vi "Configured Acquisition Trigger (Host).vi"() -> ()   [LabVIEW 2021]
doc: "Use this VI as a template to design an application that acquires data using advanced triggering logic from the NI PXIe-5170R/5171R."
uses:
  Controls/Queue_Data_Type.ctl
  <instrlib>/HSAI-RIO/Types/v1/Host/Typedefs/Temp Source.ctl
  <vilib>/FPGAPlugInAG/PXIe-5172 (8CH - 325T)/niLvFpga_Open_PXIe-5172 (8CH - 325T).vi
  <vilib>/rvi/interface/common/dynamic/niFpgaDynamicAddResources.vi
  <vilib>/FPGAPlugInAG/Dynamic/niLvFpga_Close_Dynamic.vi
  <vilib>/rvi/interface/nirviOpenFPGA/nirviOpenFPGA.xnode
  FPGA Bitfiles/Multirecord Acquisition_20220927.lvbitx
  <vilib>/rvi/interface/nirviCloseFPGA/nirviCloseFPGA.xnode
  Device Session/Device Session.lvclass
  <instrlib>/HSAI-RIO/Types/v1/Host/niHSAI Types v1 Host.lvlib
  <vilib>/Utility/TDMS File Viewer/NI_TDMS File Viewer.lvlib
panel:
  out "error out 2":errorcluster
  out "appended path":path
  out "Trigger":bool
  in  "trigger level lo (V)":dbl=-0.25
  in  "trigger level hi (V)":dbl=0.25
  out "actual sample rate":dbl=200000000.0 format="%#_6p"
  in  "onboard sample clock rate":dbl(ring)=200000000.0 items=["250 MHz"=250000000.0, "200 MHz"=200000000.0, "150 MHz"=150000000.0]
  in  "impedance":enum8{"Default", "1 mega ohm", "50 ohm"}(ring)=enum."50 ohm"
  in  "vertical offset (V)":dbl format="%.2p"
  out "Graph":T1(graph)=[{"relativeX"=-2.5e-06, "sample rate"=5e-09, "data in"=[0.6086595323350694, 0.6082560221354166, 0.606594509548611, 0.6064046223958333, 0.6059061686197916, 0.6071879069010416, 0.6087544759114583, 0.6111043294270833, 0.6109144422743055, 0.6111043294270833, 0.6073777940538194, 0.6095377604166666, 0.6135491265190971, 0.606594509548611, 0.6074727376302083, 0.610012478298611, 0.6123860677083333, 0.6079711914062499, 0.613857693142361, 0.6101311577690971, 0.6120775010850694, 0.6082560221354166, 0.6126708984374999, 0.6097276475694444, 0.6118876139322916, 0.6109144422743055, 0.6097276475694444, 0.6128607855902777, 0.6109144422743055, 0.6095377604166666, 0.6115790473090277, 0.6128607855902777, 0.6139526367187499, 0.6110093858506944, 0.609157986111111, 0.6076863606770833, 0.6129557291666666, 0.6110093858506944, 0.6092529296874999, 0.6120775010850694, 0.6131693522135416, 0.6108194986979166, 0.6126708984374999, 0.6101311577690971, 0.6068793402777777, 0.6114841037326388, 0.6140475802951388, 0.6120775010850694, 0.6108194986979166, 0.6083509657118055, 0.610226101345486, 0.6116977267795138, 0.6115790473090277, 0.6137627495659721, 0.611294216579861, 0.6116977267795138, 0.6105109320746527, 0.6104159884982638, 0.6079711914062499, 0.6094428168402777, 0.6128607855902777, 0.6097276475694444, 0.6101311577690971, 0.6093478732638888, 0.6140475802951388, 0.612575954861111, 0.6087544759114583, 0.6094428168402777, 0.6104159884982638, 0.6115790473090277, 0.6072828504774305, 0.6098225911458333, 0.608944363064236, 0.6110093858506944, 0.6075676812065971, 0.607876247829861, 0.6092529296874999, 0.6094428168402777, 0.610226101345486, 0.6118876139322916, 0.6116977267795138, 0.6086595323350694, 0.6096327039930555, 0.6072828504774305, 0.6073777940538194, 0.6075676812065971, 0.6118876139322916, 0.6074727376302083, 0.6069742838541666, 0.6045294867621527, 0.6111043294270833, 0.6067843967013888, 0.611294216579861, 0.6122911241319444, 0.6107245551215277, 0.6080661349826388, 0.6068793402777777, 0.6088494194878471, 0.6104159884982638, 0.6105109320746527, 0.6124810112847221, 0.6080661349826388, 0.6104159884982638, 0.611294216579861, 0.6111992730034721, 0.6072828504774305, 0.6110093858506944, 0.6111043294270833, 0.6119825575086805, 0.6111043294270833, 0.6110093858506944, 0.6121961805555555, 0.612575954861111, 0.6108194986979166, 0.6104159884982638, 0.6071879069010416, 0.6103210449218749, 0.6103210449218749, 0.6147359212239583, 0.6121961805555555, 0.6114841037326388, 0.6064046223958333, 0.6093478732638888, 0.6081610785590277, 0.610012478298611, 0.6083509657118055, 0.610226101345486, 0.6092529296874999, 0.6120775010850694, 0.6103210449218749, 0.6119825575086805, 0.6126708984374999, 0.6122911241319444, 0.6142374674479166, 0.6115790473090277, 0.6158989800347221, 0.6111043294270833, 0.607876247829861, 0.6103210449218749, 0.608944363064236, 0.6142374674479166, 0.6111043294270833, 0.6123860677083333, 0.609157986111111, 0.6096327039930555, 0.6071879069010416, 0.6084459092881944, 0.6116977267795138, 0.610226101345486, 0.6099175347222221, 0.6082560221354166, 0.6098225911458333, 0.6087544759114583, 0.6098225911458333, 0.6107245551215277, 0.6093478732638888, 0.6111043294270833, 0.6122911241319444, 0.610226101345486, 0.6118876139322916, 0.6081610785590277, 0.6081610785590277, 0.6082560221354166, 0.6040547688802083, 0.6075676812065971, 0.6070929633246527, 0.6083509657118055, 0.6111992730034721, 0.6106058756510416, 0.6114841037326388, 0.6104159884982638, 0.6143324110243055, 0.6117926703559027, 0.6116977267795138, 0.6123860677083333, 0.6122911241319444, 0.6105109320746527, 0.6088494194878471, 0.6123860677083333, 0.6086595323350694, 0.6127658420138888, 0.6090393066406249, 0.6109144422743055, 0.6122911241319444, 0.6094428168402777, 0.6077813042534721, 0.6071879069010416, 0.609157986111111, 0.6092529296874999, 0.6090393066406249, 0.6086595323350694, 0.6050279405381944, 0.6086595323350694, 0.6076863606770833, 0.6061197916666666, 0.606594509548611, 0.6097276475694444, 0.6101311577690971, 0.6088494194878471, 0.610012478298611, 0.6081610785590277, 0.6057162814670138, 0.6113891601562499, 0.6087544759114583, 0.6080661349826388, 0.6113891601562499, 0.6132642957899305, 0.6108194986979166, 0.6114841037326388, 0.609157986111111, 0.6077813042534721, 0.6077813042534721, 0.6146172417534721, 0.6084459092881944, 0.6111992730034721, 0.6080661349826388, 0.6088494194878471, 0.6054077148437499, 0.6085408528645833, 0.6049329969618055, 0.6075676812065971, 0.6104159884982638, 0.6104159884982638, 0.6111992730034721, 0.6096327039930555, 0.6064995659722221, 0.6051228841145833, 0.6067843967013888, 0.602962917751736, 0.6096327039930555, 0.6083509657118055, 0.6070929633246527, 0.6074727376302083, 0.6121961805555555, 0.6122911241319444, 0.6092529296874999, 0.6139526367187499, 0.6120775010850694, 0.6110093858506944, 0.6107245551215277, 0.6132642957899305, 0.607876247829861, 0.607876247829861, 0.6051228841145833, 0.6093478732638888, 0.6070929633246527, 0.6110093858506944, 0.609157986111111, 0.6084459092881944, 0.6097276475694444, 0.6155192057291666, 0.6103210449218749, 0.6086595323350694, 0.6117926703559027, 0.6099175347222221, 0.6132642957899305, 0.6084459092881944, 0.6081610785590277, 0.6067843967013888, 0.6096327039930555, 0.6114841037326388, 0.6119825575086805, 0.6075676812065971, 0.6109144422743055, 0.6129557291666666, 0.610226101345486, 0.6121961805555555, 0.6137627495659721, 0.6111043294270833, 0.609157986111111, 0.6092529296874999, 0.6109144422743055, 0.6064046223958333, 0.6070929633246527, 0.6093478732638888, 0.6097276475694444, 0.6115790473090277, 0.6118876139322916, 0.6106058756510416, 0.6135491265190971, 0.6126708984374999, 0.6079711914062499, 0.6103210449218749, 0.6101311577690971, 0.6105109320746527, 0.6120775010850694, 0.6088494194878471, 0.6097276475694444, 0.6120775010850694, 0.6080661349826388, 0.6108194986979166, 0.6123860677083333, 0.6104159884982638, 0.6120775010850694, 0.6126708984374999, 0.6094428168402777, 0.6120775010850694, 0.6115790473090277, 0.6123860677083333, 0.6104159884982638, 0.6093478732638888, 0.6097276475694444, 0.6098225911458333, 0.6056213378906249, 0.6108194986979166, 0.607876247829861, 0.6111992730034721, 0.6082560221354166, 0.6082560221354166, 0.6106058756510416, 0.608944363064236, 0.6094428168402777, 0.6071879069010416, 0.608944363064236, 0.6062147352430555, 0.6075676812065971, 0.6097276475694444, 0.6114841037326388, 0.6072828504774305, 0.608944363064236, 0.6093478732638888, 0.6084459092881944, 0.6101311577690971, 0.6056213378906249, 0.611294216579861, 0.6083509657118055, 0.6097276475694444, 0.6085408528645833, 0.6116977267795138, 0.6109144422743055, 0.6111043294270833, 0.6098225911458333, 0.613857693142361, 0.6115790473090277, 0.6121961805555555, 0.6096327039930555, 0.6124810112847221, 0.6115790473090277, 0.6116977267795138, 0.610226101345486, 0.6124810112847221, 0.6154242621527777, 0.6110093858506944, 0.6092529296874999, 0.6106058756510416, 0.608944363064236, 0.6104159884982638, 0.6085408528645833, 0.6140475802951388, 0.6097276475694444, 0.609157986111111, 0.6077813042534721, 0.6055026584201388, 0.6095377604166666, 0.6147359212239583, 0.6115790473090277, 0.6111043294270833, 0.6101311577690971, 0.6090393066406249, 0.6103210449218749, 0.611294216579861, 0.6083509657118055, 0.6143324110243055, 0.6121961805555555, 0.6111043294270833, 0.608944363064236, 0.6116977267795138, 0.6120775010850694, 0.610226101345486, 0.6145222981770833, 0.612575954861111, 0.6137627495659721, 0.6104159884982638, 0.6120775010850694, 0.6107245551215277, 0.610226101345486, 0.6134541829427083, 0.6116977267795138, 0.6153293185763888, 0.6103210449218749, 0.6118876139322916, 0.6080661349826388, 0.6124810112847221, 0.6108194986979166, 0.6118876139322916, 0.6106058756510416, 0.6106058756510416, 0.6144273546006944, 0.6127658420138888, 0.612575954861111, 0.608944363064236, 0.6111043294270833, 0.6099175347222221, 0.613644070095486, 0.6150207519531249, 0.6147359212239583, 0.613857693142361, 0.6097276475694444, 0.6118876139322916, 0.6046481662326388, 0.6111043294270833, 0.6098225911458333, 0.608944363064236, 0.607876247829861, 0.611294216579861, 0.6132642957899305, 0.611294216579861, 0.6088494194878471, 0.610226101345486, 0.6087544759114583, 0.6129557291666666, 0.6056213378906249, 0.6119825575086805, 0.6096327039930555, 0.6135491265190971, 0.6062147352430555, 0.608944363064236, 0.6101311577690971, 0.6132642957899305, 0.6090393066406249, 0.6128607855902777, 0.6093478732638888, 0.6105109320746527, 0.6064046223958333, 0.6095377604166666, 0.6085408528645833, 0.610226101345486, 0.6101311577690971, 0.6101311577690971, 0.6126708984374999, 0.6096327039930555, 0.6105109320746527, 0.6121961805555555, 0.6116977267795138, 0.6118876139322916, 0.6096327039930555, 0.6105109320746527, 0.6106058756510416, 0.6096327039930555, 0.6092529296874999, 0.6110093858506944, 0.612575954861111, 0.613644070095486, 0.6094428168402777, 0.6117926703559027, 0.610012478298611, 0.612575954861111, 0.6107245551215277, 0.6111992730034721, 0.6109144422743055, 0.6067843967013888, 0.6051228841145833, 0.6072828504774305, 0.6062147352430555, 0.6080661349826388, 0.6107245551215277, 0.6160888671874999, 0.6103210449218749, 0.6114841037326388, 0.6113891601562499, 0.6104159884982638, 0.609157986111111, 0.6092529296874999, 0.6064995659722221, 0.6106058756510416, 0.6117926703559027, 0.6117926703559027, 0.6141425238715277, 0.6099175347222221, 0.6096327039930555, 0.6127658420138888, 0.6131693522135416, 0.6105109320746527, 0.6119825575086805, 0.6128607855902777, 0.6081610785590277, 0.6085408528645833, 0.6099175347222221, 0.611294216579861, 0.610012478298611, 0.6103210449218749, 0.6071879069010416, 0.611294216579861, 0.6051228841145833, 0.6084459092881944, 0.6082560221354166, 0.6124810112847221, 0.6109144422743055, 0.6108194986979166, 0.6131693522135416, 0.6107245551215277, 0.6119825575086805, 0.6121961805555555, 0.6143324110243055, 0.6114841037326388, 0.6115790473090277, 0.6164923773871527, 0.6106058756510416, 0.6109144422743055, 0.6116977267795138, 0.6084459092881944, 0.6106058756510416, 0.6081610785590277, 0.605312771267361, 0.6081610785590277, 0.6066894531249999, 0.608944363064236, 0.607876247829861, 0.6111043294270833, 0.6109144422743055, 0.6116977267795138, 0.6137627495659721, 0.6117926703559027, 0.6099175347222221, 0.6083509657118055, 0.6094428168402777, 0.6105109320746527, 0.6085408528645833, 0.6107245551215277, 0.610226101345486, 0.6118876139322916, 0.608944363064236, 0.6123860677083333, 0.6099175347222221, 0.610226101345486, 0.6055026584201388, 0.612575954861111, 0.6115790473090277, 0.6109144422743055, 0.6079711914062499, 0.6111043294270833, 0.6072828504774305, 0.610012478298611, 0.6083509657118055, 0.611294216579861, 0.6070929633246527, 0.6119825575086805, 0.6094428168402777, 0.6123860677083333, 0.6115790473090277, 0.6113891601562499, 0.6122911241319444, 0.6099175347222221, 0.6111992730034721, 0.6108194986979166, 0.6110093858506944, 0.6084459092881944, 0.6066894531249999, 0.6057162814670138, 0.6084459092881944, 0.6116977267795138, 0.6090393066406249, 0.610226101345486, 0.6104159884982638, 0.6087544759114583, 0.6094428168402777, 0.6088494194878471, 0.6081610785590277, 0.6119825575086805, 0.6101311577690971, 0.610226101345486, 0.6079711914062499, 0.6119825575086805, 0.6092529296874999, 0.6113891601562499, 0.609157986111111, 0.6064046223958333, 0.6076863606770833, 0.6114841037326388, 0.609157986111111, 0.6116977267795138, 0.6082560221354166, 0.6097276475694444, 0.6093478732638888, 0.6132642957899305, 0.6124810112847221, 0.6123860677083333, 0.6115790473090277, 0.6152343749999999, 0.610226101345486, 0.6103210449218749, 0.6081610785590277, 0.6095377604166666, 0.6054077148437499, 0.6068793402777777, 0.606594509548611, 0.612575954861111, 0.6058112250434027, 0.6124810112847221, 0.6048380533854166, 0.612575954861111, 0.6095377604166666, 0.6135491265190971, 0.6095377604166666, 0.612575954861111, 0.6106058756510416, 0.6117926703559027, 0.6121961805555555, 0.6117926703559027, 0.6086595323350694, 0.6104159884982638, 0.610012478298611, 0.609157986111111, 0.6093478732638888, 0.6111043294270833, 0.6081610785590277, 0.6088494194878471, 0.6088494194878471, 0.6077813042534721, 0.6070929633246527, 0.605312771267361, 0.6068793402777777, 0.6118876139322916, 0.6097276475694444, 0.6116977267795138, 0.6073777940538194, 0.610012478298611, 0.6072828504774305, 0.6090393066406249, 0.6052178276909721, 0.6084459092881944, 0.604244656032986, 0.6098225911458333, 0.6103210449218749, 0.610012478298611, 0.6104159884982638, 0.6134541829427083, 0.6114841037326388, 0.6140475802951388, 0.6126708984374999, 0.607876247829861, 0.6103210449218749, 0.6132642957899305, 0.6106058756510416, 0.6113891601562499, 0.6064995659722221, 0.6111043294270833, 0.6099175347222221, 0.6099175347222221, 0.6094428168402777, 0.6144273546006944, 0.6113891601562499, 0.611294216579861, 0.6124810112847221, 0.6123860677083333, 0.6152343749999999, 0.6124810112847221, 0.6121961805555555, 0.6115790473090277, 0.6141425238715277, 0.6096327039930555, 0.6107245551215277, 0.6081610785590277, 0.6098225911458333, 0.6099175347222221, 0.6057162814670138, 0.6074727376302083, 0.6086595323350694, 0.6123860677083333, 0.6122911241319444, 0.6122911241319444, 0.6103210449218749, 0.6101311577690971, 0.6050279405381944, 0.6057162814670138, 0.608944363064236, 0.6116977267795138, 0.6064995659722221, 0.6126708984374999, 0.606594509548611, 0.608944363064236, 0.606594509548611, 0.6114841037326388, 0.6087544759114583, 0.6093478732638888, 0.6087544759114583, 0.6095377604166666, 0.6064995659722221, 0.6120775010850694, 0.6103210449218749, 0.6147359212239583, 0.6122911241319444, 0.6110093858506944, 0.6088494194878471, 0.6081610785590277, 0.6074727376302083, 0.608944363064236, 0.6055026584201388, 0.6145222981770833, 0.6116977267795138, 0.6123860677083333, 0.610226101345486, 0.6114841037326388, 0.6121961805555555, 0.6135491265190971, 0.6095377604166666, 0.6082560221354166, 0.6067843967013888, 0.610012478298611, 0.6075676812065971, 0.6133592393663194, 0.610012478298611, 0.6145222981770833, 0.6126708984374999, 0.6143324110243055, 0.6122911241319444, 0.6093478732638888, 0.6062147352430555, 0.6059061686197916, 0.6033664279513888, 0.6051228841145833, 0.6071879069010416, 0.6094428168402777, 0.611294216579861, 0.6101311577690971, 0.6095377604166666, 0.6087544759114583, 0.6115790473090277, 0.6147359212239583, 0.6104159884982638, 0.6131693522135416, 0.610012478298611, 0.6081610785590277, 0.6067843967013888, 0.6087544759114583, 0.6061197916666666, 0.6084459092881944, 0.6104159884982638, 0.6119825575086805, 0.6111992730034721, 0.6105109320746527, 0.6086595323350694, 0.6086595323350694, 0.6098225911458333, 0.6111992730034721, 0.6076863606770833, 0.6132642957899305, 0.6084459092881944, 0.6096327039930555, 0.6086595323350694, 0.6124810112847221, 0.607876247829861, 0.6088494194878471, 0.6092529296874999, 0.6123860677083333, 0.6109144422743055, 0.6114841037326388, 0.6126708984374999, 0.6106058756510416, 0.6092529296874999, 0.6084459092881944, 0.6072828504774305, 0.6086595323350694, 0.6062147352430555, 0.6115790473090277, 0.6127658420138888, 0.6150207519531249, 0.6126708984374999, 0.614925808376736, 0.6139526367187499, 0.615993923611111, 0.6079711914062499, 0.6122911241319444, 0.6107245551215277, 0.6153293185763888, 0.6120775010850694, 0.611294216579861, 0.6111992730034721, 0.6130506727430555, 0.6116977267795138, 0.6097276475694444, 0.6066894531249999, 0.6093478732638888, 0.6087544759114583, 0.610012478298611, 0.6098225911458333, 0.6131693522135416, 0.6123860677083333, 0.6124810112847221, 0.6087544759114583, 0.6095377604166666, 0.6077813042534721, 0.6076863606770833, 0.6060011121961805, 0.610012478298611, 0.610012478298611, 0.6103210449218749, 0.6142374674479166, 0.6153293185763888, 0.616207546657986, 0.6110093858506944, 0.6132642957899305, 0.6129557291666666, 0.611294216579861, 0.6103210449218749, 0.6098225911458333, 0.6113891601562499, 0.6094428168402777, 0.6098225911458333, 0.6111992730034721, 0.6128607855902777, 0.6128607855902777, 0.611294216579861, 0.6123860677083333, 0.6127658420138888, 0.6094428168402777, 0.6068793402777777, 0.6068793402777777, 0.6107245551215277, 0.6083509657118055, 0.613644070095486, 0.607876247829861, 0.6115790473090277, 0.6097276475694444, 0.6109144422743055, 0.6101311577690971, 0.6115790473090277, 0.6145222981770833, 0.6116977267795138, 0.6062147352430555, 0.6086595323350694, 0.6107245551215277, 0.6098225911458333, 0.6145222981770833, 0.6119825575086805, 0.6148308648003471, 0.6113891601562499, 0.6070929633246527, 0.6067843967013888, 0.6062147352430555, 0.6090393066406249, 0.6079711914062499, 0.6090393066406249, 0.6101311577690971, 0.6130506727430555, 0.6116977267795138, 0.6103210449218749, 0.6079711914062499, 0.6067843967013888, 0.6086595323350694, 0.6090393066406249, 0.6087544759114583, 0.6090393066406249, 0.6104159884982638, 0.6083509657118055, 0.6124810112847221, 0.6110093858506944, 0.6107245551215277, 0.6120775010850694, 0.6090393066406249, 0.6090393066406249, 0.6099175347222221, 0.6103210449218749, 0.6073777940538194, 0.611294216579861, 0.6086595323350694, 0.6103210449218749, 0.6121961805555555, 0.6109144422743055, 0.6087544759114583, 0.610012478298611, 0.6045294867621527, 0.6064995659722221, 0.6036512586805555, 0.6101311577690971, 0.6092529296874999, 0.6107245551215277, 0.6092529296874999, 0.6148308648003471, 0.6101311577690971, 0.6092529296874999, 0.6062147352430555, 0.6069742838541666, 0.6090393066406249, 0.6070929633246527, 0.6111043294270833, 0.6101311577690971, 0.6114841037326388, 0.6147359212239583, 0.6148308648003471, 0.6143324110243055, 0.6135491265190971, 0.6122911241319444, 0.6106058756510416, 0.6115790473090277, 0.6114841037326388, 0.6130506727430555, 0.6094428168402777, 0.608944363064236, 0.6101311577690971, 0.6077813042534721, 0.6093478732638888, 0.6122911241319444, 0.6094428168402777, 0.6145222981770833, 0.6093478732638888, 0.610012478298611, 0.6114841037326388, 0.6109144422743055, 0.6104159884982638, 0.610226101345486, 0.6097276475694444, 0.6093478732638888, 0.6117926703559027, 0.6146172417534721, 0.610012478298611, 0.611294216579861, 0.6110093858506944, 0.6127658420138888, 0.6131693522135416, 0.6104159884982638, 0.6129557291666666, 0.6095377604166666, 0.6069742838541666, 0.6118876139322916, 0.6093478732638888, 0.6099175347222221, 0.6120775010850694, 0.6119825575086805, 0.6139526367187499, 0.6084459092881944, 0.6092529296874999, 0.6116977267795138, 0.6070929633246527, 0.6086595323350694, 0.610012478298611, 0.6087544759114583, 0.6064046223958333, 0.6108194986979166, 0.6069742838541666, 0.6139526367187499, 0.6088494194878471, 0.6108194986979166, 0.6143324110243055, 0.613644070095486, 0.6088494194878471, 0.6123860677083333, 0.6110093858506944, 0.6153293185763888, 0.6076863606770833, 0.6103210449218749, 0.607876247829861, 0.6119825575086805, 0.6077813042534721, 0.6116977267795138, 0.6106058756510416, 0.6137627495659721, 0.6113891601562499, 0.6093478732638888, 0.6062147352430555, 0.6093478732638888, 0.6123860677083333, 0.6104159884982638, 0.6124810112847221, 0.6155192057291666, 0.613857693142361, 0.6114841037326388, 0.6098225911458333, 0.6127658420138888, 0.6086595323350694, 0.6085408528645833, 0.6054077148437499, 0.6104159884982638, 0.6064995659722221, 0.611294216579861, 0.6092529296874999, 0.612575954861111, 0.6134541829427083, 0.6097276475694444, 0.6099175347222221, 0.6108194986979166, 0.6097276475694444, 0.614925808376736, 0.6132642957899305, 0.6154242621527777, 0.6142374674479166, 0.6120775010850694, 0.6118876139322916, 0.6128607855902777, 0.611294216579861, 0.6103210449218749, 0.6072828504774305, 0.6105109320746527, 0.6058112250434027, 0.607876247829861, 0.6148308648003471, 0.6115790473090277, 0.6101311577690971, 0.6106058756510416, 0.6074727376302083, 0.6107245551215277, 0.6127658420138888, 0.6098225911458333, 0.6095377604166666, 0.6088494194878471, 0.6113891601562499, 0.6153293185763888, 0.6110093858506944, 0.6119825575086805, 0.6080661349826388]}, ...(2 in all)]
  out "fpga temperature (°C)":dbl(slide)=84.16040039062506 scale=0.0..96.0 scale format="%#_6p"
  out "power consumption (W)":dbl(slide)=28.75 scale=0.0..38.25 scale format="%#_6p"
  in  "decimation factor":u16=1
  in  "coupling":enum8{"Default", "DC", "AC"}(ring)
  in  "bandwidth":T2(ring)
  in  "pretrigger samples":u64=500
  in  "number of samples":u64=1000
  in  "RIO Device":tag="PXI1Slot2"
  in  "channel(s)":string="0,1"
  in  "vertical range (Vpp)":dbl=1.0 format="%.2p"
  out "error out":errorcluster
  in  "stop":bool
  # "RIO Device"
  # "Vertical Settings"
  # "Trigger Settings"
  # "System Monitor"
  # "Acquisition Settings"
  # "Clocking"
  # "DSP"
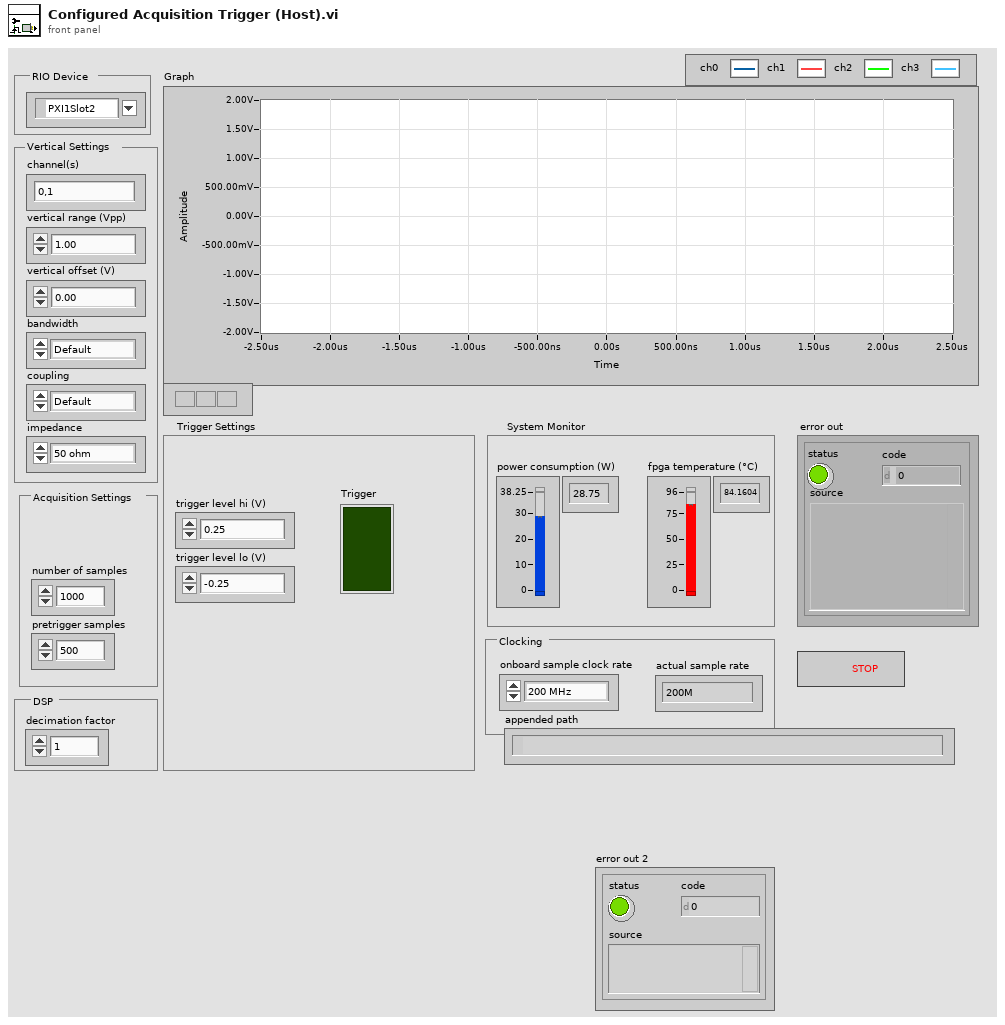
[diagram p1: front panel]
types:
  T1 = cluster{"relativeX":dbl, "sample rate":dbl, "data in":dbl[]}[]
  T2 = enum8{"Default", "Full Bandwidth", "Anti-alias Filter", "80 MHz FIR Filter", "40 MHz FIR Filter", "20 MHz FIR Filter"}
  T3 = enum16{"Immediate", "A", "B", "OR", "AND", "A THEN B", "B THEN A", "High Resolution"}
  T4 = typedef "niHSAI Types v1 Host.lvlib/Temp Source.ctl" = enum8{"Device Temperature", "Thermal Shutdown Margin", "FPGA Temperature", "FPGA Temperature Limit"}
  T5 = typedef "Queue_Data_Type.ctl" = cluster{"date/time string":string, "data":dbl[][]}
  T6 = enum16{"open", "open or create", "create or replace", "create", "open (read-only)"}
  T7 = cluster{"date/time string":string, "data":dbl[][]}
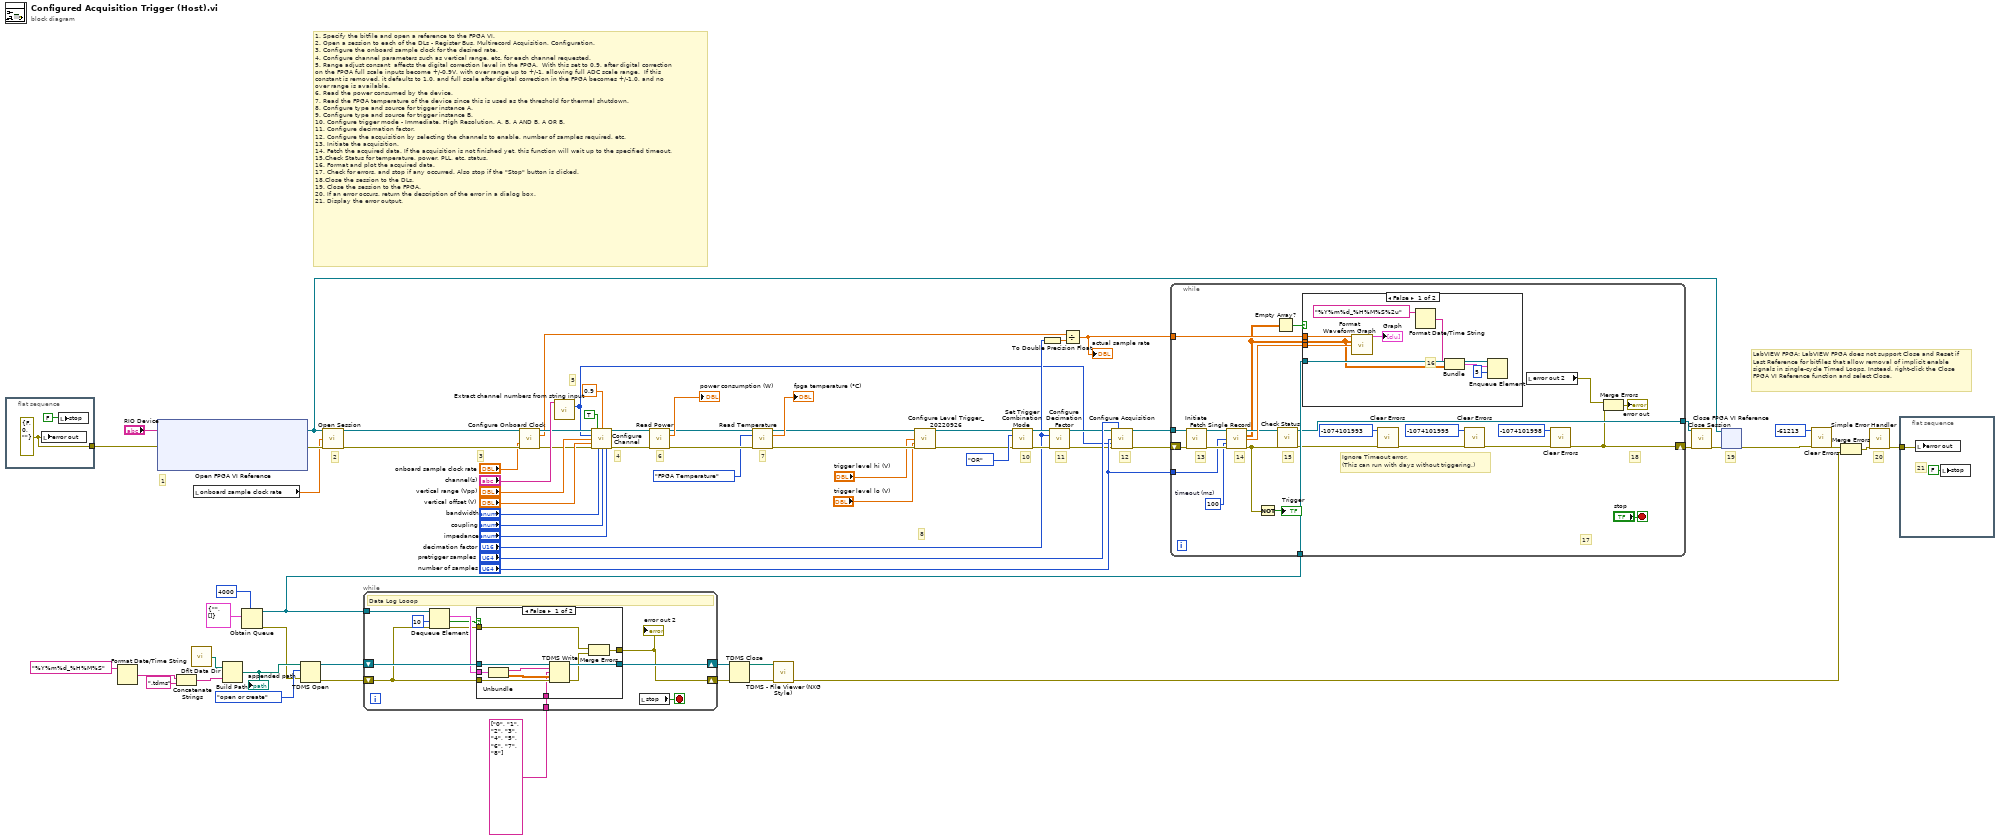
[diagram p0: block diagram]
diagram:
  # "4"
  # "5"
  # "7"
  # "6"
  # "11"
  # "3"
  # "10"
  # "8"
  # "12"
  # "LabVIEW FPGA: LabVIEW FPGA does not support Close and Reset if Last Reference for bitfiles that allow removal of implicit enable signals in single-cycle Timed Loops. Instead, right-click the Close FPGA VI Reference function and select Close."
  # "20"
  # "19"
  # "1. Specify the bitfile and open a reference to the FPGA VI.\n2. Open a session to each of the DLs - Register Bus, Multirecord Acquisition, Configuration.\n3. Configure the onboard sample clock for the desired rate.\n4. Configure channel parameters such as vertical range, etc. for each channel requested.\n5. Range adjust consant  affects the digital correction level in the FPGA.  With this set to 0.9, after digital correction\non the FPGA full scale inputs become +/-0.9V, with over range up to +/-1, allowing full ADC scale range.  If this \nconstant is removed, it defaults to 1.0, and full scale after digital correction in the FPGA becomes +/-1.0, and no\nover range is available.  \n6. Read the power consumed by the device.\n7. Read the FPGA temperature of the device since this is used as the threshold for thermal shutdown.\n8. Configure type and source for trigger instance A.\n9. Configure type and source for trigger instance B.\n10. Configure trigger mode - Immediate, High Resolution, A, B, A AND B, A OR B.\n11. Configure decimation factor.\n12. Configure the acquisition by selecting the channels to enable, number of samples required, etc.\n13. Initiate the acquisition.\n14. Fetch the acquired data. If the acquisition is not finished yet, this function will wait up to the specified timeout.\n15.Check Status for temperature, power, PLL, etc. status. \n16. Format and plot the acquired data.\n17. Check for errors, and stop if any occurred. Also stop if the \"Stop\" button is clicked.\n18.Close the session to the DLs.\n19. Close the session to the FPGA.\n20. If an error occurs, return the description of the error in a dialog box.\n21. Display the error output."
  # "2"
  # "1"
  n1 = flat-sequence {
    tunnel: [w74] -> w65
    frame #0 {
      w74 = errorcluster {"status"=FALSE, "code"=0, "source"=""} ("error out")
      n2 = local write "error out"(w74) -> ()
      n3 = local write "stop"(FALSE ("stop")) -> ()
    }
  }
  n4 = Format Date/Time String(time format string (%c)="%Y%m%d_%H%M%S") -> (date/time string=w63:string)  [unwired: 2 in]
  n5 = xnode "Open FPGA VI Reference"("error in"=w65, "resource name"="RIO Device") -> ("FPGA VI Reference Out"=w68:refnum<k20>, "error out"=w69:errorcluster)
  n6 = Concatenate Strings(w63, ".tdms" ("string")) -> (w62:string)
  n7 = call <vilib>:"Dflt Data Dir.vi"() -> ("App:Default Data Directory"=w64:path)
  n8 = local read "onboard sample clock rate"() -> (w67:dbl)
  n9 = Build Path(base path=w64, name or relative path=w62) -> (appended path=w59:path)
  "appended path" <- w59
  n10 = Obtain Queue(max queue size (-1, unlimited)=4000, element data type=T5 {"date/time string"="", "data"=[]} ("cluster")) -> (queue out=w49:refnum<queue>, error out=w57:errorcluster)  [unwired: 3 in, 1 out]
  n11 = TDMS Open(8:w57, 10:T6."open or create" ("operation (0:open)"), 11:w59) -> (0:w55:errorcluster, 3:w52:refnum<k34>)  [unwired: 4 in]
  n12 = call "Open Session.vi"("fpga reference in"=w68, "adc clock rate (Hz)"=w67, "error in"=w69) -> ("device session out"=w72:refnum<class "Device Session.lvclass">, "error out"=w71:errorcluster)  [unwired: 11 in]
  n13 = while {
    shift-right: [w77] -> w54
    shift-left: w55 -> [w82]
    shift-right: [w84] -> w51
    shift-left: w52 -> [w85]
    tunnel: w49 -> [w83]
    tunnel: string[] ["0", "1", "2", "3", "4", "5", "6", "7", "8"] ("channel name(s) in (Untitled)") -> [w75]
    stop <- w79 stop-if-true
    # "Data Log Looop"
    n14 = Dequeue Element(queue=w83, timeout in ms (-1)=10, error in (no error)=w82) -> (element=w81:T5, timed out?=w76:bool, error out=w80:errorcluster)  [unwired: 1 out]
    n15 = case shown="False" w76 {
      tunnel: w85 -> [w95 w97]
      tunnel: [w94 w97] -> w84
      tunnel: w82 -> [w93 _]
      tunnel: w81 -> [w92 _]
      tunnel: w80 -> [w91 w96]
      tunnel: [w89 w96] -> w77
      tunnel: w75 -> [w86 _]
      frame False {
        n16 = Unbundle(w92) -> ("date/time string"=w88:string, "data"=w87:dbl[][])
        n17 = TDMS Write(0:w95, 5:w88, 7:w86, 9:w87, 11:w93) -> (4:w94:refnum<k34>, 15:w90:errorcluster)  [unwired: 1 in, 2 out]
        n18 = Merge Errors(w91, w90) -> (w89:errorcluster)
      }
      frame True {
        # "Timed out. No data."
      }
    }
    "error out 2" <- w77
    n19 = local read "stop"() -> (w79:bool)
  }
  n20 = call "Configure Onboard Clock.vi"("device session in"=w72, "adc clock rate (Hz)"="onboard sample clock rate", "error in"=w71) -> ("device session out"=w34:refnum<class "Device Session.lvclass">, "actual adc clock rate (Hz)"=w26:dbl, "error out"=w33:errorcluster)  [unwired: 9 in, 1 out]
  n21 = call "Extract channel numbers from string input.vi"("channel input"="channel(s)") -> ("array of chans"=w8:u32[])  [unwired: 13 in, 1 out]
  n22 = call "Configure Channel.vi"("device session in"=w34, "enable channel (T)"=TRUE ("enable channel"), "range adjust"=0.9, "channels"=w8, "vertical range (Vpp)"="vertical range (Vpp)", "vertical offset (V)"="vertical offset (V)", "error in"=w33, "bandwidth"="bandwidth", "coupling"="coupling", "impedance"="impedance") -> ("device session out"=w20:refnum<class "Device Session.lvclass">, "error out"=w19:errorcluster)  [unwired: 4 in]
  n23 = call "Read Power.vi"("device session in"=w20, "error in"=w19) -> ("device session out"=w21:refnum<class "Device Session.lvclass">, "power (W)"=→"power consumption (W)":dbl, "error out"=w22:errorcluster)  [unwired: 11 in]
  n24 = TDMS Close(8:w54, 11:w51) -> (0:w53:errorcluster, 3:w50:path)
  n25 = call "Read Temperature.vi"("device session in"=w21, "source"=Temp_Source."FPGA Temperature", "error in"=w22) -> ("device session out"=w18:refnum<class "Device Session.lvclass">, "temperature (°C)"=→"fpga temperature (°C)":dbl, "error out"=w17:errorcluster)  [unwired: 10 in]
  n26 = call <vilib>:"TDMS - File Viewer (NXG Style).vi"("error in"=w53, "file in"=w50) -> ("error out"=w47:errorcluster)  [unwired: 8 in, 1 out]
  n27 = call "Configure Level Trigger_20220926.vi"("device session in"=w18, "trigger level hi (V)"="trigger level hi (V)", "trigger level lo (V)"="trigger level lo (V)", "error in"=w17) -> ("device session out"=w7:refnum<class "Device Session.lvclass">, "error out"=w6:errorcluster)  [unwired: 10 in]
  n28 = call "Set Trigger Combination Mode.vi"("device session in"=w7, "mode"=T3."OR", "error in"=w6) -> ("device session out"=w31:refnum<class "Device Session.lvclass">, "error out"=w30:errorcluster)  [unwired: 11 in]
  n29 = To Double Precision Float(number="decimation factor") -> (double precision float=w32:dbl)
  n30 = call "Configure Decimation Factor.vi"("device session in"=w31, "decimation factor"="decimation factor", "error in"=w30) -> ("device session out"=w28:refnum<class "Device Session.lvclass">, "error out"=w29:errorcluster)  [unwired: 11 in]
  n31 = Divide(x=w26, y=w32) -> (x/y=w10:dbl)
  "actual sample rate" <- w10
  n32 = call "Configure Acquisition.vi"("device session in"=w28, "pretrigger samples"="pretrigger samples", "number of samples"="number of samples", "channels to store"=w8, "error in"=w29) -> ("device session out"=w39:refnum<class "Device Session.lvclass">, "error out"=w40:errorcluster)  [unwired: 8 in, 1 out]
  n33 = while {
    tunnel: w49 -> [w122]
    tunnel: w39 -> [w118]
    tunnel: "number of samples" -> [w116]
    tunnel: w10 -> [w112]
    shift-right: [w98] -> w1
    shift-left: w40 -> [w121]
    tunnel: [w99] -> w3
    stop <- "stop" stop-if-true
    w117 = 100  # timeout (ms)
    # "Ignore Timeout error.\n(This can run with days without triggering.)"
    # "15"
    # "17"
    # "14"
    # "13"
    # "18"
    n34 = call "Initiate.vi"("device session in"=w118, "error in"=w121) -> ("device session out"=w119:refnum<class "Device Session.lvclass">, "error out"=w120:errorcluster)  [unwired: 12 in]
    n35 = call "Fetch Single Record.vi"("device session in"=w119, "number of samples"=w116, "timeout (ms)"=w117, "error in"=w120) -> ("device session out"=w113:refnum<class "Device Session.lvclass">, "data"=w104:dbl[][], "relativeX (samples)"=w115:dbl, "error out"=w105:errorcluster)  [unwired: 7 in, 1 out]
    n36 = Not(x=w105) -> (.not. x?=→"Trigger":bool)
    n37 = Empty Array?(array=w104) -> (empty?=w103:bool)
    n38 = call "Check Status.vi"("device session in"=w113, "error in"=w105) -> ("device session out"=w99:refnum<class "Device Session.lvclass">, "error out"=w114:errorcluster)  [unwired: 12 in]
    n39 = case shown="False" w103 {
      tunnel: w104 -> [w127 _]
      tunnel: w115 -> [w131 _]
      tunnel: w112 -> [w129 _]
      tunnel: w122 -> [w128 _]
      frame False {
        # "16"
        n40 = call "Format Waveform Graph.vi"("sample rate (Hz)"=w129, "data in"=w127, "relativeX (samples)"=w131) -> ("waveform out"=→"Graph":T1)  [unwired: 12 in]
        n41 = Format Date/Time String(time format string (%c)="%Y%m%d_%H%M%S%2u") -> (date/time string=w123:string)  [unwired: 2 in]
        n42 = Bundle("date/time string"=w123, "data"=w127) -> (w124:T7)  [unwired: 1 in]
        n43 = Enqueue Element(queue=w128, element=w124, timeout in ms (-1)=5) -> ()  [unwired: 1 in, 3 out]
      }
      frame True {
        # "No data"
      }
    }
    n44 = call <vilib>:"Clear Errors.vi"("error in (no error)"=w114, "specific error code to clear (0: all)"=-1074101993) -> ("error out"=w109:errorcluster)  [unwired: 4 in, 1 out]
    n45 = call <vilib>:"Clear Errors.vi"("error in (no error)"=w109, "specific error code to clear (0: all)"=-1074101995) -> ("error out"=w107:errorcluster)  [unwired: 4 in, 1 out]
    n46 = local read "error out 2"() -> (w101:errorcluster)
    n47 = call <vilib>:"Clear Errors.vi"("error in (no error)"=w107, "specific error code to clear (0: all)"=-1074101998) -> ("error out"=w98:errorcluster)  [unwired: 4 in, 1 out]
    n48 = Merge Errors(w101, w98) -> (→"error out":errorcluster)
  }
  n49 = call "Close Session.vi"("device session in"=w3, "error in"=w1) -> ("error out"=w2:errorcluster)  [unwired: 13 in]
  n50 = xnode "Close FPGA VI Reference"("FPGA VI Reference In"=w68, "error in"=w2) -> ("error out"=w43:errorcluster)
  n51 = call <vilib>:"Clear Errors.vi"("error in (no error)"=w43, "specific error code to clear (0: all)"=-61213) -> ("error out"=w42:errorcluster)  [unwired: 4 in, 1 out]
  n52 = Merge Errors(w42, w47) -> (w48:errorcluster)
  n53 = call <vilib>:"Simple Error Handler.vi"("error in (no error)"=w48) -> ("error out"=w66:errorcluster)  [unwired: 4 in, 4 out]
  n54 = flat-sequence {
    tunnel: w66 -> [w133]
    frame #0 {
      # "21"
      n55 = local write "error out"(w133) -> ()
      n56 = local write "stop"(FALSE ("stop")) -> ()
    }
  }
